vi "IMAQdx_AbsImage_Flea3_v4.4.vi"() -> ()   [LabVIEW 2012]
doc: "Take a single PixelFly exposure and display the result as an intensity graph.This VI illustrates the basics of taking an exposure with the PixelFly camera. Use Ctrl-H to get help on any of the controls\n\nCopyright 2001, The Cooke Corporation."
uses:
  LabVIEW Data V4.10/Shared Libraries/Controls/FileName_Cluster.ctl
  <vilib>/userdefined/High Color/IMAQdx.ctl
  <vilib>/vision/driver/IMAQdx.llb/IMAQdx Acquisition Mode.ctl
  Shared Libraries/Controls/FileInfo_Global.vi
  <vilib>/vision/driver/NI_Vision_Acquisition_Software.lvlib
panel:
  out "DDE Done":bool=TRUE
  out "Waiting for PIXIS file":bool=TRUE
  in  "Flea Acquire":bool=TRUE
  in  "PIXIS Acquire":bool=TRUE
  out "PIXIS Loop":i32
  out "CycleDone":bool
  out "PIXIS Frames":i64
  in  "Interrupt":bool
  out "Status":string="Running..."
  in  "stop":bool
  in  "Tab Control":enum32{"Setup", "Images", "Hardware status"}(tab)=enum."Images"
  in  "PIXIS Data Series Name":string="Sr_PIXIS_Seq"
  in  "Flea File Parameters":T1={"Data Root"=path "C:/Experiment/Data", "Index"=4, "Instrument"="Flea3_20S4M"} {"Index" format="%04d"}
  in  "PIXIS Wave Name":string="Test_Img"
  out "PIXIS Image Note":string="Experiment=Sr\nCamera_ID=PIXIS\nImageType=Raw\nDataType=Absorption\nImageDirection=XY\nMagnification=5.480000E+0\nFileNumber=4\nIndex=0\nIndexedWaves=BlueLaserLockOffset;DipPowX;DipPowX2;DipPowZ;DoppCoolDet;DoppCoolSweep;Nspacers;Pdet;TOF;TOFaux;Xshim;Yshim;ZshimVar;bLoadT;bMapT;combWidthI;dopCoolT;freq;holdT;loadT;rMOTbroadDetuningF;rMOTbroadDetuningI;rMOTpow2;rMOTpow3;rMOTpow4;singleFreqDet;varWaveP1\nIndexedValues=525.000000000000E-3;3.00000000000000E+0;3.00000000000000E+0;250.000000000000E-3;-1.78000000000000E+3;20.0000000000000E+0;4.00000000000000E+0;600.000000000000E-3;25.0000000000000E-3;18.0000000000000E-3;350.000000000000E-3;875.000000000000E-3;1.52200000000000E+0;5.40000000000000E+0;400.000000000000E-6;2.25000000000000E+0;20.0000000000000E-3;3.00000000000000E+3;500.000000000000E-3;35.0000000000000E-3;2.22500000000000E+0;2.45000000000000E+0;1.60000000000000E+0;1.35000000000000E+0;1.30000000000000E+0;-1.57500000000000E+3;3.50000000000000E+0\n# Current Variables\n#\nholdT = 5.000000E-1\nBlueLaserLockOffset = 5.250000E-1\nDipPowX = 3.000000E+0\nDipPowX2 = 3.000000E+0\nDipPowXLat = 1.500000E+0\nDipPowZ = 2.500000E-1\nDipPowZ2 = 2.500000E-2\nDipPowZ3 = 2.500000E-2\nDoppCoolDet = -1.780000E+3\nDoppCoolSweep = 2.000000E+1\nHeatingAmp = 1.000000E-1\nMOTPow = 8.000000E+0\nMOTcurrent = -7.500000E+0\nMOTdetuning = -4.500000E+1\nNspacers = 4.000000E+0\nPdet = 6.000000E-1\nPdet2 = 5.000000E-2\nProbeDet = 0.000000E+0\nProbePow = 2.000000E+0\nTOF = 2.500000E-2\nTOFaux = 1.800000E-2\nXshim = 3.500000E-1\nYshim = 8.750000E-1\nZshim = 1.600000E+0\nZshimVar = 1.522000E+0\nbLoadT = 5.400000E+0\nbMapT = 4.000000E-4\ncombWidthF = 1.500000E-1\ncombWidthI = 2.250000E+0\ncompensation = -3.981000E+0\ndopCoolT = 2.000000E-2\ndopCoolT1 = 1.500000E-2\nfreq = 3.000000E+3\nloadT = 3.500000E-2\nminus_zman = -7.904000E+0\nplus_zman = -9.792000E+0\nrMOTbroadDetuningF = 2.225000E+0\nrMOTbroadDetuningI = 2.450000E+0\nrMOTcurrF = -2.000000E-1\nrMOTcurrI = -2.000000E-1\nrMOTpow1 = 7.000000E+0\nrMOTpow2 = 1.600000E+0\nrMOTpow3 = 1.350000E+0\nrMOTpow4 = 1.300000E+0\nsingleFreqDet = -1.575000E+3\ntEvap0 = 1.000000E-1\ntEvap1 = 2.000000E+0\ntEvap2 = 3.000000E-1\ntau = 6.000000E-1\nvarWaveP1 = 3.500000E+0\nvarWaveP2 = 3.500000E+0\n#\n# Master Staging List\n#Comment\tMarker\tMode\tGroup\tDelay\tX ODT Shuttter\tX ODT AO TTL\tY ODT Shutter\tY ODT AO TTL\tZ ODT Shutter\tZ ODT AO TTL\t707 Shutter\tPB_7\tPB_8\tFreq Switch rMOT\trMOT AO TTL\t\tTrans AO TTL\tProbe AO TTL\tZman AO TTL\tbMOT AO TTL\t60 Hz Trig Gate\tWindow Heater TTL\tPB_18\tPB_19\tPB_20 Trigger Dev3\tPB_21 Trigger Dev2\tPB_22 Trigger Dev1\tPB_23 Trigger Dev0\tStep\t~Atomic Beam Shutter\tGate Valve\tDO0_2\tDO0_3\t~Zman Coils\t~ MOT Coils\t~ Dipole Flea3 Shutter\trMOT Shutter\t+Zeeman Coils\t-Zeeman Coils\tCompensation Coils\tMOT Coils\trMOT AO Power\trMOT Freq Amplitude\trMOT Freq Offset\tAO0_7\tTrans Shutter\tProbe Shutter\tZman Shutter\tbMOT Shutter\tDO1_4\t679 Shutter\t~ Pixis Shutter\t~Abs Flea3 Shutter\tMOT AO Frequency\tMOT AO Power\tProbe AO Power\tProbe AO Frequency\tX Shim Coils\tY Shim Coils\tZ Shim Coils\tZ ODT AO Power\tPIXIS Ext Shutter\tD02_1\tD02_2\tD02_3\tD02_4\tD02_5\tD02_6\tD02_7\tAO2_0\tAO2_1\tD03_0\tD03_1\tD03_2\tD03_3\tD03_4\tD03_5\tD03_6\tD03_7\tAO3_0\tAO3_1\tAO3_2\tVariable Waveplate\t461 Spec Offset\tAO3_5\tAO3_6\tX ODT AO Power\tSRS Freq\tSRS Amp\tSRS Offset\tSRS Func Type\tRedMotDDS\tRedMotDDS_ 0\tRedMotDDS_ 1\tRedMotDDS_ 2\r\n\r\nreset\t\tRamp\t1\t.1\t1\t1\t0\t0\t0\t1\t1\t0\t0\t0\t1\t0\t1\t1\t1\t0\t0\t0\t0\t0\t0\t0\t0\t0\t0\t0\t1\t0\t0\t0\t0\t1\t0\tplus_zman\tminus_zman\tcompensation\tMOTcurrent\trMOTpow1\tcombAmplitude(combWidthI)\trMOTdelta(-(rMOTbroadDetuningI +combWidthI/2))\t0\t1\t0\t1\t1\t0\t1\t1\t1\tbMOTdelta(MOTdetuning)\tbMOTpow(0.5)\tProbePow\tPdet2\tXshim\tYshim\tZshim\tODTpowY(DipPowZ)\t0\t0\t0\t0\t0\t0\t0\t0\t0\t0\t0\t0\t0\t0\t0\t0\t0\t0\t0\t0\t0\tvarWaveP1\tBlueLaserLockOffset\t0\t0\tODTpowX(DipPowX)\tfreq\tHeatingAmp\t0\tSine\tDetuning\tsingleFreqDet\t-20\t8\r\nblue MOT load\t\tRamp\t1\tbLoadT\t1\t1\t0\t0\t0\t1\t0\t0\t0\t0\t1\t0\t1\t1\t1\t1\t0\t0\t0\t0\t0\t0\t0\t0\t0\t0\t1\t0\t0\t0\t0\t1\t0\tplus_zman\tminus_zman\tcompensation\tMOTcurrent\trMOTpow1\tcombAmplitude(combWidthI)\trMOTdelta(-(rMOTbroadDetuningI +combWidthI/2))\t0\t1\t0\t1\t1\t0\t0\t1\t1\tbMOTdelta(MOTdetuning)\tbMOTpow(MOTPow)\tProbePow\tPdet2\tXshim\tYshim\tZshim\tODTpowY(DipPowZ)\t0\t0\t0\t0\t0\t0\t0\t0\t0\t0\t0\t0\t0\t0\t0\t0\t0\t0\t0\t0\t0\tvarWaveP1\tBlueLaserLockOffset\t0\t0\tODTpowX(DipPowX)\tfreq\tHeatingAmp\t0\tSine\tDetuning\tsingleFreqDet\t-20\t8\r\npretrig\t\tRamp\t1\t6.244e-3\t1\t1\t0\t0\t0\t1\t0\t0\t0\t0\t1\t0\t1\t1\t1\t1\t0\t1\t0\t0\t0\t0\t0\t0\t0\t0\t1\t0\t0\t0\t0\t0\t0\tplus_zman\tminus_zman\tcompensation\tMOTcurrent\trMOTpow1\tcombAmplitude(combWidthI)\trMOTdelta(-(rMOTbroadDetuningI +combWidthI/2))\t0\t1\t0\t1\t1\t0\t0\t0\t0\tbMOTdelta(MOTdetuning)\tbMOTpow(MOTPow)\tProbePow\tPdet2\tXshim\tYshim\tZshim\tODTpowY(DipPowZ)\t0\t0\t0\t0\t0\t0\t0\t0\t0\t0\t0\t0\t0\t0\t0\t0\t0\t0\t0\t0\t0\tvarWaveP1\tBlueLaserLockOffset\t0\t0\tODTpowX(DipPowX)\tfreq\tHeatingAmp\t0\tSine\tDetuning\tsingleFreqDet\t-20\t8\r\nCamWaitTime\t\tRamp\t1\t0.275\t1\t1\t0\t0\t0\t1\t0\t0\t0\t0\t1\t0\t1\t1\t1\t1\t0\t1\t0\t0\t0\t0\t0\t0\t0\t0\t1\t0\t0\t0\t0\t1\t0\tplus_zman\tminus_zman\tcompensation\tMOTcurrent\trMOTpow1\tcombAmplitude(combWidthI)\trMOTdelta(-(rMOTbroadDetuningI +combWidthI/2))\t0\t1\t0\t1\t1\t0\t0\t1\t1\tbMOTdelta(MOTdetuning)\tbMOTpow(MOTPow)\tProbePow\tPdet2\tXshim\tYshim\tZshim\tODTpowZ(DipPowZ)\t0\t0\t0\t0\t0\t0\t0\t0\t0\t0\t0\t0\t0\t0\t0\t0\t0\t0\t0\t0\t0\tvarWaveP1\tBlueLaserLockOffset\t0\t0\tODTpowX(DipPowX)\tfreq\tHeatingAmp\t0\tSine\tDetuning\tsingleFreqDet\t-20\t8\r\nProbeShutOn\t\tRamp\t1\t1120e-6\t1\t1\t0\t0\t0\t1\t0\t0\t0\t0\t1\t0\t1\t1\t1\t1\t0\t1\t0\t0\t0\t0\t0\t0\t0\t0\t1\t0\t0\t0\t0\t1\t1\tplus_zman\tminus_zman\tcompensation\tMOTcurrent\trMOTpow1\tcombAmplitude(combWidthI)\trMOTdelta(-(rMOTbroadDetuningI +combWidthI/2))\t0\t1\t0\t1\t1\t0\t0\t1\t1\tbMOTdelta(MOTdetuning)\tbMOTpow(MOTPow)\tProbePow\tPdet2\tXshim\tYshim\tZshim\tODTpowZ(DipPowZ)\t0\t0\t0\t0\t0\t0\t0\t0\t0\t0\t0\t0\t0\t0\t0\t0\t0\t0\t0\t0\t0\tvarWaveP1\tBlueLaserLockOffset\t0\t0\tODTpowX(DipPowX)\tfreq\tHeatingAmp\t0\tSine\tDetuning\tsingleFreqDet\t-20\t8\r\nRepumpShutOff\t\tRamp\t1\t260e-6\t1\t1\t0\t0\t0\t1\t0\t0\t0\t0\t1\t0\t1\t1\t1\t1\t0\t1\t0\t0\t0\t0\t0\t0\t0\t0\t1\t0\t0\t0\t0\t1\t1\tplus_zman\tminus_zman\tcompensation\tMOTcurrent\trMOTpow1\tcombAmplitude(combWidthI)\trMOTdelta(-(rMOTbroadDetuningI +combWidthI/2))\t0\t1\t0\t0\t1\t0\t0\t1\t1\tbMOTdelta(MOTdetuning)\tbMOTpow(MOTPow)\tProbePow\tPdet2\tXshim\tYshim\tZshim\tODTpowZ(DipPowZ)\t0\t0\t0\t0\t0\t0\t0\t0\t0\t0\t0\t0\t0\t0\t0\t0\t0\t0\t0\t0\t0\tvarWaveP1\tBlueLaserLockOffset\t0\t0\tODTpowX(DipPowX)\tfreq\tHeatingAmp\t0\tSine\tDetuning\tsingleFreqDet\t-20\t8\r\nMOTShutOff\t\tRamp\t1\t1370e-6\t1\t1\t0\t0\t0\t1\t1\t0\t0\t0\t1\t0\t1\t1\t1\t1\t0\t1\t0\t0\t0\t0\t0\t0\t0\t0\t1\t0\t0\t0\t0\t1\t1\tplus_zman\tminus_zman\tcompensation\tMOTcurrent\trMOTpow1\tcombAmplitude(combWidthI)\trMOTdelta(-(rMOTbroadDetuningI +combWidthI/2))\t0\t1\t0\t0\t0\t0\t1\t1\t1\tbMOTdelta(MOTdetuning)\tbMOTpow(MOTPow)\tProbePow\tPdet2\tXshim\tYshim\tZshim\t0\t0\t0\t0\t0\t0\t0\t0\t0\t0\t0\t0\t0\t0\t0\t0\t0\t0\t0\t0\t0\t0\tvarWaveP1\tBlueLaserLockOffset\t0\t0\tODTpowX(DipPowX)\tfreq\tHeatingAmp\t0\tSine\tDetuning\tsingleFreqDet\t-20\t8\r\nCoil Switch\t\tRamp\t1\t220e-6\t1\t1\t0\t0\t0\t0\t1\t0\t0\t0\t1\t0\t1\t1\t0\t0\t0\t1\t0\t0\t0\t0\t0\t0\t0\t0\t1\t0\t0\t0\t0\t1\t1\tplus_zman\tminus_zman\tcompensation\trMOTcurrI\trMOTpow1\tcombAmplitude(combWidthI)\trMOTdelta(-(rMOTbroadDetuningI +combWidthI/2))\t0\t1\t0\t0\t0\t0\t1\t1\t1\tbMOTdelta(MOTdetuning)\tbMOTpow(0.5)\tProbePow\tPdet2\tXshim\tYshim\tZshim\t0\t0\t0\t0\t0\t0\t0\t0\t0\t0\t0\t0\t0\t0\t0\t0\t0\t0\t0\t0\t0\t0\tvarWaveP1\tBlueLaserLockOffset\t0\t0\tODTpowX(DipPowX)\tfreq\tHeatingAmp\t0\tSine\tDetuning\tsingleFreqDet\t-20\t8\r\n60HzTrigger\t\tHalt\t1\t10u\t1\t1\t0\t0\t0\t0\t1\t0\t0\t0\t1\t0\t1\t1\t0\t0\t1\t1\t0\t0\t0\t0\t0\t0\t0\t0\t1\t0\t0\t0\t0\t1\t1\tplus_zman\tminus_zman\tcompensation\trMOTcurrI\trMOTpow1\tcombAmplitude(combWidthI)\trMOTdelta(-(rMOTbroadDetuningI +combWidthI/2))\t0\t1\t0\t0\t0\t0\t1\t1\t1\tbMOTdelta(MOTdetuning)\tbMOTpow(0.5)\tProbePow\tPdet2\tXshim\tYshim\tZshim\t0\t0\t0\t0\t0\t0\t0\t0\t0\t0\t0\t0\t0\t0\t0\t0\t0\t0\t0\t0\t0\t0\tvarWaveP1\tBlueLaserLockOffset\t0\t0\tODTpowX(DipPowX)\tfreq\tHeatingAmp\t0\tSine\tDetuning\tsingleFreqDet\t-20\t8\r\nCapture Red MOT\t\tRamp\t1\t.1\t1\t1\t0\t0\t0\t0\t1\t0\t0\t0\t1\t0\t0\t1\t0\t0\t0\t1\t0\t0\t0\t0\t0\t0\t0\t0\t1\t0\t0\t0\t0\t1\t1\tplus_zman\tminus_zman\tcompensation\trMOTcurrI\trMOTpow1\tcombAmplitude(combWidthI)\trMOTdelta(-(rMOTbroadDetuningI +combWidthI/2))\t0\t1\t0\t0\t0\t0\t1\t1\t1\tbMOTdelta(MOTdetuning)\tbMOTpow(0.5)\tProbePow\tPdet2\tXshim\tYshim\tZshim\tODTpowZ(DipPowZ)\t0\t0\t0\t0\t0\t0\t0\t0\t0\t0\t0\t0\t0\t0\t0\t0\t0\t0\t0\t0\t0\tvarWaveP1\tBlueLaserLockOffset\t0\t0\tODTpowX(DipPowX)\tfreq\tHeatingAmp\t0\tSine\tDetuning\tsingleFreqDet\t-20\t8\r\nRamp Red MOT\t\tRamp\t1\t.4\t1\t1\t0\t0\t0\t0\t1\t0\t0\t0\t1\t0\t0\t1\t0\t0\t0\t1\t0\t0\t0\t0\t0\t0\t10u\t0\t1\t0\t0\t0\t0\t1\t1\tplus_zman\tminus_zman\tcompensation\trMOTcurrI\tHalfGaussRamp(t,rMOTpow1,rMOTpow2, .4)\tLineRamp(f,combAmplitude(combWidthI),combAmplitude(combWidthF))\tLineRamp(f,rMOTdelta(-(rMOTbroadDetuningI +combWidthI/2)),rMOTdelta(-(rMOTbroadDetuningF +combWidthF/2)))\t0\t1\t0\t0\t0\t0\t1\t1\t1\tbMOTdelta(MOTdetuning)\tbMOTpow(0.5)\tProbePow\tPdet2\tXshim\tYshim\tLineRamp(f,Zshim,ZshimVar)\tODTpowZ(DipPowZ)\t0\t0\t0\t0\t0\t0\t0\t0\t0\t0\t0\t0\t0\t0\t0\t0\t0\t0\t0\t0\t0\tvarWaveP1\tLineRamp(f,BlueLaserLockOffset,Pdet)\t0\t0\tODTpowX(DipPowX)\tfreq\tHeatingAmp\t0\tSine\tDetuning\tsingleFreqDet\t-20\t8\r\nSF\t\tRamp\t1\t.07\t1\t1\t0\t0\t0\t0\t0\t0\t0\t1\t1\t0\t0\t1\t0\t0\t0\t1\t0\t0\t0\t0\t0\t0\t10u\t0\t1\t0\t0\t0\t0\t1\t1\tplus_zman\tminus_zman\tcompensation\trMOTcurrI\tLineRamp(f,rMOTpow2,rMOTpow3)\tcombAmplitude(combWidthF)\trMOTdelta(-(rMOTbroadDetuningF +combWidthF/2))\t0\t1\t0\t0\t0\t0\t0\t1\t1\tbMOTdelta(MOTdetuning)\tbMOTpow(0.5)\tProbePow\tPdet2\tXshim\tYshim\tZshimVar\tODTpowZ(DipPowZ)\t0\t0\t0\t0\t0\t0\t0\t0\t0\t0\t0\t0\t0\t0\t0\t0\t0\t0\t0\t0\t0\tvarWaveP1\tPdet\t0\t0\tODTpowX(DipPowX)\tfreq\tHeatingAmp\t0\tSine\tDetuning\tsingleFreqDet\t-20\t8\r\nload1\t\tRamp\t1\tloadT\t1\t1\t0\t0\t0\t0\t0\t0\t0\t1\t1\t0\t0\t1\t0\t0\t0\t1\t0\t0\t0\t0\t0\t0\t0\t0\t1\t0\t0\t0\t0\t1\t1\tplus_zman\tminus_zman\tcompensation\trMOTcurrI\trMOTpow3\tcombAmplitude(combWidthF)\trMOTdelta(-(rMOTbroadDetuningF +combWidthF/2))\t0\t1\t0\t0\t0\t0\t0\t1\t1\tbMOTdelta(MOTdetuning)\tbMOTpow(0.5)\tProbePow\tPdet2\tXshim\tYshim\tZshimVar\tODTpowZ(DipPowZ)\t0\t0\t0\t0\t0\t0\t0\t0\t0\t0\t0\t0\t0\t0\t0\t0\t0\t0\t0\t0\t0\tvarWaveP1\tPdet\t0\t0\tODTpowX(DipPowX)\tfreq\tHeatingAmp\t0\tSine\tDetuning\tsingleFreqDet\t-20\t8\r\nload2\t\tRamp\t0\t.05\t1\t1\t0\t0\t0\t0\t0\t0\t0\t1\t1\t0\t0\t1\t0\t0\t0\t1\t0\t0\t0\t0\t0\t0\t0\t0\t1\t0\t0\t0\t0\t1\t1\tplus_zman\tminus_zman\tcompensation\trMOTcurrI\trMOTpow3\tcombAmplitude(combWidthF)\trMOTdelta(-(rMOTbroadDetuningF +combWidthF/2))\t0\t1\t0\t0\t0\t0\t0\t1\t1\tbMOTdelta(MOTdetuning)\tbMOTpow(0.5)\tProbePow\tPdet2\tXshim\tYshim\tZshimVar\tODTpowZ(DipPowZ)\t0\t0\t0\t0\t0\t0\t0\t0\t0\t0\t0\t0\t0\t0\t0\t0\t0\t0\t0\t0\t0\tvarWaveP1\tPdet\t0\t0\tODTpowX(DipPowX)\tfreq\tHeatingAmp\t0\tSine\tDetuning\tsingleFreqDet\t-20\t8\r\ndrop Red MOT\t\tRamp\t1\t.05\t1\t1\t0\t0\t0\t0\t0\t0\t0\t1\t0\t0\t0\t1\t0\t0\t0\t1\t0\t0\t0\t0\t0\t0\t0\t0\t1\t0\t0\t0\t1\t1\t0\tplus_zman\tminus_zman\tcompensation\trMOTcurrF\trMOTpow3\tcombAmplitude(combWidthF)\trMOTdelta(-(rMOTbroadDetuningF +combWidthF/2))\t0\t1\t0\t0\t0\t0\t0\t1\t1\tbMOTdelta(MOTdetuning)\tbMOTpow(0.5)\tProbePow\tPdet2\tXshim\tYshim\tZshimVar\tODTpowZ(DipPowZ)\t0\t0\t0\t0\t0\t0\t0\t0\t0\t0\t0\t0\t0\t0\t0\t0\t0\t0\t0\t0\t0\tvarWaveP1\tPdet\t0\t0\tODTpowX(DipPowX)\tfreq\tHeatingAmp\t0\tSine\tDetuning\tsingleFreqDet\t-20\t8\r\nramp Trap\t\tRamp\t0\t.05\t1\t1\t0\t0\t0\t0\t0\t0\t0\t1\t0\t0\t0\t1\t0\t0\t0\t1\t0\t0\t0\t0\t0\t0\t10u\t0\t1\t0\t0\t0\t1\t1\t0\tplus_zman\tminus_zman\tcompensation\trMOTcurrF\trMOTpow3\tcombAmplitude(combWidthF)\trMOTdelta(-(rMOTbroadDetuningF +combWidthF/2))\t0\t1\t0\t0\t0\t0\t0\t1\t1\tbMOTdelta(MOTdetuning)\tbMOTpow(0.5)\tProbePow\tPdet2\tXshim\tYshim\tZshimVar\tODTpowZ(DipPowZ)\t0\t0\t0\t0\t0\t0\t0\t0\t0\t0\t0\t0\t0\t0\t0\t0\t0\t0\t0\t0\t0\tvarWaveP1\tPdet\t0\t0\tSinRamp(t,(ODTpowX(DipPowX)+ODTpowX(DipPowX2))/2,(ODTpowX(DipPowX2)-ODTpowX(DipPowX))/2,10,3*pi/2)\tfreq\tHeatingAmp\t0\tSine\tDetuning\tsingleFreqDet\t-20\t8\r\nhold\t\tRamp\t0\t.01\t1\t1\t0\t0\t0\t0\t0\t0\t0\t1\t0\t0\t0\t1\t0\t0\t0\t1\t0\t0\t0\t0\t0\t0\t0\t0\t1\t0\t0\t0\t1\t1\t1\tplus_zman\tminus_zman\tcompensation\trMOTcurrF\trMOTpow4\tcombAmplitude(combWidthF)\trMOTdelta(-(rMOTbroadDetuningF +combWidthF/2))\t0\t1\t0\t0\t0\t0\t0\t1\t1\tbMOTdelta(MOTdetuning)\tbMOTpow(0.5)\tProbePow\tPdet2\tXshim\tYshim\tZshimVar\tODTpowZ(DipPowZ)\t0\t0\t0\t0\t0\t0\t0\t0\t0\t0\t0\t0\t0\t0\t0\t0\t0\t0\t0\t0\t0\tvarWaveP1\tPdet\t0\t0\tODTpowX(DipPowX2)\tfreq\tHeatingAmp\t0\tSine\tDetuning\tDoppCoolDet\t-20\t8\r\nDoppler Cool1\t\tRamp\t0\tdopCoolT\t1\t1\t0\t0\t0\t0\t0\t0\t0\t1\t1\t0\t0\t1\t0\t0\t0\t1\t0\t0\t0\t0\t0\t0\t10u\t0\t1\t0\t0\t0\t1\t1\t1\tplus_zman\tminus_zman\tcompensation\trMOTcurrF\trMOTpow4\tcombAmplitude(combWidthF)\trMOTdelta(-(rMOTbroadDetuningF +combWidthF/2))\t0\t0\t0\t0\t0\t0\t0\t1\t1\tbMOTdelta(MOTdetuning)\tbMOTpow(0.5)\tProbePow\tPdet2\tXshim\tYshim\tZshimVar\tODTpowZ(DipPowZ)\t0\t0\t0\t0\t0\t0\t0\t0\t0\t0\t0\t0\t0\t0\t0\t0\t0\t0\t0\t0\t0\tvarWaveP1\tPdet\t0\t0\tODTpowX(DipPowX2)\tfreq\tHeatingAmp\t0\tSine\tDetuning\tDoppCoolDet\t-20\t8\r\nDoppler Cool2\t\tRamp\t0\tdopCoolT\t1\t1\t0\t0\t0\t0\t0\t0\t0\t1\t1\t0\t0\t1\t0\t0\t0\t1\t0\t0\t0\t0\t0\t0\t10u\t0\t1\t0\t0\t0\t1\t1\t1\tplus_zman\tminus_zman\tcompensation\trMOTcurrF\trMOTpow4\tcombAmplitude(combWidthF)\trMOTdelta(-(rMOTbroadDetuningF +combWidthF/2))\t0\t0\t0\t0\t0\t0\t0\t1\t1\tbMOTdelta(MOTdetuning)\tbMOTpow(0.5)\tProbePow\tPdet2\tXshim\tYshim\tZshimVar\tODTpowZ(DipPowZ)\t0\t0\t0\t0\t0\t0\t0\t0\t0\t0\t0\t0\t0\t0\t0\t0\t0\t0\t0\t0\t0\tvarWaveP1\tPdet\t0\t0\tODTpowX(DipPowX2)\tfreq\tHeatingAmp\t0\tSine\tRamp\tDoppCoolDet\tDoppCoolDet-DoppCoolSweep\tdopCoolT*1000\r\nDoppler Cool3\t\tRamp\t0\tdopCoolT\t1\t1\t0\t0\t0\t0\t0\t0\t0\t1\t1\t0\t0\t1\t0\t0\t0\t1\t0\t0\t0\t0\t0\t0\t10u\t0\t1\t0\t0\t0\t1\t1\t1\tplus_zman\tminus_zman\tcompensation\trMOTcurrF\trMOTpow4\tcombAmplitude(combWidthF)\trMOTdelta(-(rMOTbroadDetuningF +combWidthF/2))\t0\t0\t0\t0\t0\t0\t0\t1\t1\tbMOTdelta(MOTdetuning)\tbMOTpow(0.5)\tProbePow\tPdet2\tXshim\tYshim\tZshimVar\tODTpowZ(DipPowZ)\t0\t0\t0\t0\t0\t0\t0\t0\t0\t0\t0\t0\t0\t0\t0\t0\t0\t0\t0\t0\t0\tvarWaveP1\tPdet\t0\t0\tODTpowX(DipPowX2)\tfreq\tHeatingAmp\t0\tSine\tDetuning\tDoppCoolDet-DoppCoolSweep\tDoppCoolDet-DoppCoolSweep\tdopCoolT*1000\r\nhold\t\tRamp\t0\tholdT\t1\t1\t0\t0\t0\t0\t0\t0\t0\t1\t0\t0\t0\t1\t0\t0\t0\t1\t0\t0\t0\t0\t0\t0\t0\t0\t1\t0\t0\t0\t1\t1\t0\tplus_zman\tminus_zman\tcompensation\trMOTcurrF\trMOTpow4\tcombAmplitude(combWidthF)\trMOTdelta(-(rMOTbroadDetuningF +combWidthF/2))\t0\t1\t0\t0\t0\t0\t0\t1\t1\tbMOTdelta(MOTdetuning)\tbMOTpow(0.5)\tProbePow\tPdet2\tXshim\tYshim\tZshimVar\tODTpowZ(DipPowZ)\t0\t0\t0\t0\t0\t0\t0\t0\t0\t0\t0\t0\t0\t0\t0\t0\t0\t0\t0\t0\t0\tvarWaveP1\tPdet\t0\t0\tODTpowX(DipPowX2)\tfreq\tHeatingAmp\t0\tSine\tDetuning\tDoppCoolDet-DoppCoolSweep\tDoppCoolDet-DoppCoolSweep\tdopCoolT*1000\r\ndrop HTrap\t\tRamp\t0\t.03\t1\t1\t0\t0\t1\t1\t1\t0\t0\t1\t0\t0\t0\t1\t0\t0\t0\t1\t0\t0\t0\t0\t0\t0\t0\t0\t1\t0\t0\t0\t0\t1\t0\tplus_zman\tminus_zman\tcompensation\trMOTcurrF\trMOTpow3\tcombAmplitude(combWidthF)\trMOTdelta(-(rMOTbroadDetuningF +combWidthF/2))\t0\t1\t0\t0\t0\t0\t1\t1\t1\tbMOTdelta(MOTdetuning)\tbMOTpow(0.5)\tProbePow\tPdet2\tXshim\tYshim\tZshimVar\tODTpowZ(DipPowZ)\t0\t0\t0\t0\t0\t0\t0\t0\t0\t0\t0\t0\t0\t0\t0\t0\t0\t0\t0\t0\t0\tvarWaveP1\tPdet\t0\t0\tODTpowX(DipPowX)\tfreq\tHeatingAmp\t0\tSine\tDetuning\tsingleFreqDet\tDoppCoolDet-DoppCoolSweep\tdopCoolT*1000\r\nmodulate\t\tRamp\t0\t3m\t1\t1\t0\t0\t1\t1\t1\t0\t0\t1\t0\t0\t0\t1\t0\t0\t0\t1\t0\t0\t0\t0\t0\t0\t0\t0\t1\t0\t0\t0\t0\t1\t0\tplus_zman\tminus_zman\tcompensation\trMOTcurrF\trMOTpow3\tcombAmplitude(combWidthF)\trMOTdelta(-(rMOTbroadDetuningF +combWidthF/2))\t0\t1\t0\t0\t0\t0\t1\t1\t1\tbMOTdelta(MOTdetuning)\tbMOTpow(0.5)\tProbePow\tPdet2\tXshim\tYshim\tZshimVar\tODTpowZ(DipPowZ)\t0\t0\t0\t0\t0\t0\t0\t0\t0\t0\t0\t0\t0\t0\t0\t0\t0\t0\t0\t0\t0\tvarWaveP1\tPdet\t0\t0\tODTpowX(DipPowX)\tfreq\tHeatingAmp\t0\tSine\tDetuning\tsingleFreqDet\tDoppCoolDet-DoppCoolSweep\tdopCoolT*1000\r\nEvaporation\t\tRamp\t0\ttEvap1\t1\t1\t0\t0\t1\t1\t1\t0\t0\t1\t0\t0\t0\t1\t0\t0\t0\t1\t0\t0\t0\t0\t0\t0\t1m\t0\t1\t0\t0\t0\t0\t1\t0\tplus_zman\tminus_zman\tcompensation\trMOTcurrF\trMOTpow3\tcombAmplitude(combWidthF)\trMOTdelta(-(rMOTbroadDetuningF +combWidthF/2))\t0\t1\t0\t0\t0\t0\t1\t1\t1\tbMOTdelta(MOTdetuning)\tbMOTpow(0.5)\tProbePow\tPdet2\tXshim\tYshim\tZshimVar\tODTpowZ(DipPowZ)\t0\t0\t0\t0\t0\t0\t0\t0\t0\t0\t0\t0\t0\t0\t0\t0\t0\t0\t0\t0\t0\tvarWaveP1\tPdet\t0\t0\tExpRamp2(t,0,ODTpowX(DipPowX),ODTpowX(DipPowX2),tau)\tfreq\tHeatingAmp\t0\tSine\tDetuning\tsingleFreqDet\tDoppCoolDet-DoppCoolSweep\tdopCoolT*1000\r\ndrop\t\tRamp\t0\t.01\t1\t1\t0\t0\t1\t1\t1\t0\t0\t1\t0\t0\t0\t1\t0\t0\t0\t1\t0\t0\t0\t0\t0\t0\t0\t0\t1\t0\t0\t0\t0\t1\t0\tplus_zman\tminus_zman\tcompensation\trMOTcurrF\trMOTpow3\tcombAmplitude(combWidthF)\trMOTdelta(-(rMOTbroadDetuningF +combWidthF/2))\t0\t1\t0\t0\t0\t0\t1\t1\t1\tbMOTdelta(MOTdetuning)\tbMOTpow(0.5)\tProbePow\tPdet2\tXshim\tYshim\tZshimVar\tODTpowZ(DipPowZ)\t0\t0\t0\t0\t0\t0\t0\t0\t0\t0\t0\t0\t0\t0\t0\t0\t0\t0\t0\t0\t0\tvarWaveP2\tPdet\t0\t0\tODTpowX(DipPowXLat)\tfreq\tHeatingAmp\t0\tSine\tDetuning\tsingleFreqDet\tDoppCoolDet-DoppCoolSweep\tdopCoolT*1000\r\nband map\t\tRamp\t0\tbMapT\t1\t1\t0\t0\t1\t1\t1\t0\t0\t1\t0\t0\t0\t1\t0\t0\t0\t1\t0\t0\t0\t0\t0\t0\t2u\t0\t1\t0\t0\t0\t0\t1\t0\tplus_zman\tminus_zman\tcompensation\trMOTcurrF\trMOTpow3\tcombAmplitude(combWidthF)\trMOTdelta(-(rMOTbroadDetuningF +combWidthF/2))\t0\t1\t0\t0\t0\t0\t1\t1\t1\tbMOTdelta(MOTdetuning)\tbMOTpow(0.5)\tProbePow\tPdet2\tXshim\tYshim\tZshimVar\tLineRamp(f,ODTpowZ(DipPowZ),ODTpowZ(-0.2))\t0\t0\t0\t0\t0\t0\t0\t0\t0\t0\t0\t0\t0\t0\t0\t0\t0\t0\t0\t0\t0\tvarWaveP2\tPdet\t0\t0\tLineRamp(f,ODTpowX(DipPowX),0)\tfreq\tHeatingAmp\t0\tSine\tDetuning\tsingleFreqDet\tDoppCoolDet-DoppCoolSweep\tdopCoolT*1000\r\nband map delay\t\tRamp\t0\t10u\t1\t1\t0\t0\t1\t1\t1\t0\t0\t1\t0\t0\t0\t1\t0\t0\t0\t1\t0\t0\t0\t0\t0\t0\t0\t0\t1\t0\t0\t0\t0\t1\t0\tplus_zman\tminus_zman\tcompensation\trMOTcurrF\trMOTpow3\tcombAmplitude(combWidthF)\trMOTdelta(-(rMOTbroadDetuningF +combWidthF/2))\t0\t1\t0\t0\t0\t0\t1\t1\t1\tbMOTdelta(MOTdetuning)\tbMOTpow(0.5)\tProbePow\tPdet2\tXshim\tYshim\tZshimVar\tODTpowZ(DipPowZ)\t0\t0\t0\t0\t0\t0\t0\t0\t0\t0\t0\t0\t0\t0\t0\t0\t0\t0\t0\t0\t0\tvarWaveP2\tPdet\t0\t0\tODTpowX(DipPowXLat)\tfreq\tHeatingAmp\t0\tSine\tDetuning\tsingleFreqDet\tDoppCoolDet-DoppCoolSweep\tdopCoolT*1000\r\nTOF\t\tRamp\t1\tTOFaux\t0\t0\t0\t0\t0\t0\t1\t0\t0\t1\t0\t0\t0\t0\t0\t0\t0\t1\t0\t0\t0\t0\t0\t0\t0\t0\t1\t0\t0\t0\t1\t1\t0\tplus_zman\tminus_zman\tcompensation\trMOTcurrF\trMOTpow4\tcombAmplitude(combWidthF)\trMOTdelta(-(rMOTbroadDetuningF +combWidthF/2))\t0\t1\t1\t0\t0\t0\t1\t1\t1\tbMOTdelta(MOTdetuning)\tbMOTpow(0.5)\tProbePow\tPdet\tXshim\tYshim\tZshimVar\tODTpowZ(DipPowZ)\t1\t0\t0\t0\t0\t0\t0\t0\t0\t0\t0\t0\t0\t0\t0\t0\t0\t0\t0\t0\t0\tvarWaveP2\tPdet\t0\t0\tODTpowX(DipPowX2)\tfreq\tHeatingAmp\t0\tSine\tDetuning\tsingleFreqDet\tDoppCoolDet-DoppCoolSweep\tdopCoolT*1000\r\nTOF\t\tRamp\t1\t.007\t0\t0\t0\t0\t0\t0\t1\t0\t0\t1\t0\t0\t0\t0\t0\t0\t0\t1\t0\t0\t0\t0\t0\t0\t0\t0\t1\t0\t0\t0\t1\t1\t0\tplus_zman\tminus_zman\tcompensation\trMOTcurrF\trMOTpow4\tcombAmplitude(combWidthF)\trMOTdelta(-(rMOTbroadDetuningF +combWidthF/2))\t0\t1\t1\t0\t0\t0\t1\t1\t1\tbMOTdelta(MOTdetuning)\tbMOTpow(0.5)\tProbePow\tPdet\tXshim\tYshim\tZshimVar\tODTpowZ(DipPowZ)\t1\t0\t0\t0\t0\t0\t0\t0\t0\t0\t0\t0\t0\t0\t0\t0\t0\t0\t0\t0\t0\tvarWaveP2\tPdet\t0\t0\tODTpowX(DipPowX2)\tfreq\tHeatingAmp\t0\tSine\tDetuning\tsingleFreqDet\tDoppCoolDet-DoppCoolSweep\tdopCoolT*1000\r\narm FLEA\t\tRamp\t1\t.000044\t0\t0\t0\t0\t0\t0\t1\t0\t0\t1\t0\t0\t0\t0\t0\t0\t0\t0\t0\t0\t0\t0\t0\t0\t0\t0\t1\t0\t0\t0\t1\t0\t0\tplus_zman\tminus_zman\tcompensation\trMOTcurrF\trMOTpow3\tcombAmplitude(combWidthF)\trMOTdelta(-(rMOTbroadDetuningF +combWidthF/2))\t0\t1\t1\t0\t0\t0\t1\t1\t0\tbMOTdelta(MOTdetuning)\tbMOTpow(0.5)\tProbePow\tPdet\tXshim\tYshim\tZshimVar\tODTpowZ(0)\t1\t0\t0\t0\t0\t0\t0\t0\t0\t0\t0\t0\t0\t0\t0\t0\t0\t0\t0\t0\t0\tvarWaveP2\tPdet\t0\t0\tODTpowX(DipPowX)\tfreq\tHeatingAmp\t0\tSine\tDetuning\tsingleFreqDet\tDoppCoolDet-DoppCoolSweep\tdopCoolT*1000\r\natom img\t\tRamp\t1\t10e-6\t0\t0\t0\t0\t0\t0\t1\t0\t0\t1\t0\t0\t0\t1\t0\t0\t0\t0\t0\t0\t0\t0\t0\t0\t0\t0\t1\t0\t0\t0\t1\t0\t0\tplus_zman\tminus_zman\tcompensation\trMOTcurrF\trMOTpow3\tcombAmplitude(combWidthF)\trMOTdelta(-(rMOTbroadDetuningF +combWidthF/2))\t0\t1\t1\t0\t0\t0\t1\t0\t0\tbMOTdelta(MOTdetuning)\tbMOTpow(0.5)\tProbePow\tPdet\tXshim\tYshim\tZshimVar\tODTpowZ(0)\t1\t0\t0\t0\t0\t0\t0\t0\t0\t0\t0\t0\t0\t0\t0\t0\t0\t0\t0\t0\t0\tvarWaveP2\tPdet\t0\t0\tODTpowX(DipPowX)\tfreq\tHeatingAmp\t0\tSine\tDetuning\tsingleFreqDet\tDoppCoolDet-DoppCoolSweep\tdopCoolT*1000\r\natom img\t\tRamp\t0\t2.8e-3\t0\t0\t0\t0\t0\t0\t1\t0\t0\t1\t0\t0\t0\t0\t0\t0\t0\t0\t0\t0\t0\t0\t0\t0\t0\t0\t1\t0\t0\t0\t1\t1\t0\tplus_zman\tminus_zman\tcompensation\trMOTcurrF\trMOTpow3\tcombAmplitude(combWidthF)\trMOTdelta(-(rMOTbroadDetuningF +combWidthF/2))\t0\t1\t1\t0\t0\t0\t1\t1\t1\tbMOTdelta(MOTdetuning)\tbMOTpow(0.5)\tProbePow\tPdet\tXshim\tYshim\tZshimVar\tODTpowZ(DipPowZ)\t1\t0\t0\t0\t0\t0\t0\t0\t0\t0\t0\t0\t0\t0\t0\t0\t0\t0\t0\t0\t0\tvarWaveP2\tPdet\t0\t0\tODTpowX(DipPowX)\tfreq\tHeatingAmp\t0\tSine\tDetuning\tsingleFreqDet\tDoppCoolDet-DoppCoolSweep\tdopCoolT*1000\r\ntransmit img\t\tRamp\t1\t.28\t0\t0\t0\t0\t0\t0\t1\t0\t0\t1\t0\t0\t0\t0\t0\t0\t0\t0\t0\t0\t0\t0\t0\t0\t0\t0\t1\t0\t0\t0\t1\t1\t0\tplus_zman\tminus_zman\tcompensation\trMOTcurrF\trMOTpow3\tcombAmplitude(combWidthF)\trMOTdelta(-(rMOTbroadDetuningF +combWidthF/2))\t0\t1\t1\t0\t0\t0\t1\t1\t1\tbMOTdelta(MOTdetuning)\tbMOTpow(0.5)\tProbePow\tPdet\tXshim\tYshim\tZshimVar\tODTpowZ(DipPowZ)\t1\t0\t0\t0\t0\t0\t0\t0\t0\t0\t0\t0\t0\t0\t0\t0\t0\t0\t0\t0\t0\tvarWaveP2\tPdet\t0\t0\tODTpowX(DipPowX)\tfreq\tHeatingAmp\t0\tSine\tDetuning\tsingleFreqDet\tDoppCoolDet-DoppCoolSweep\tdopCoolT*1000\r\narm PIXIS\t\tRamp\t1\t.007\t1\t1\t0\t0\t0\t1\t1\t0\t0\t1\t1\t0\t0\t0\t1\t1\t0\t0\t0\t0\t0\t0\t0\t0\t0\t0\t1\t0\t0\t0\t1\t1\t0\tplus_zman\tminus_zman\tcompensation\trMOTcurrF\trMOTpow1\tcombAmplitude(combWidthF)\trMOTdelta(-(rMOTbroadDetuningF +combWidthF/2))\t0\t1\t1\t0\t0\t0\t1\t1\t1\tbMOTdelta(MOTdetuning)\tbMOTpow(0.5)\tProbePow\tPdet\tXshim\tYshim\tZshimVar\tODTpowZ(DipPowZ)\t1\t0\t0\t0\t0\t0\t0\t0\t0\t0\t0\t0\t0\t0\t0\t0\t0\t0\t0\t0\t0\tvarWaveP2\tPdet\t0\t0\tODTpowX(DipPowX)\tfreq\tHeatingAmp\t0\tSine\tDetuning\tsingleFreqDet\tDoppCoolDet-DoppCoolSweep\tdopCoolT*1000\r\narm FLEA\t\tRamp\t1\t44e-6\t1\t1\t0\t0\t0\t1\t1\t0\t0\t1\t1\t0\t0\t0\t1\t1\t0\t0\t0\t0\t0\t0\t0\t0\t0\t0\t1\t0\t0\t0\t1\t0\t0\tplus_zman\tminus_zman\tcompensation\trMOTcurrF\trMOTpow1\tcombAmplitude(combWidthF)\trMOTdelta(-(rMOTbroadDetuningF +combWidthF/2))\t0\t1\t1\t0\t0\t0\t1\t1\t0\tbMOTdelta(MOTdetuning)\tbMOTpow(0.5)\tProbePow\tPdet\tXshim\tYshim\tZshimVar\tODTpowZ(DipPowZ)\t1\t0\t0\t0\t0\t0\t0\t0\t0\t0\t0\t0\t0\t0\t0\t0\t0\t0\t0\t0\t0\tvarWaveP2\tPdet\t0\t0\tODTpowX(DipPowX)\tfreq\tHeatingAmp\t0\tSine\tDetuning\tsingleFreqDet\tDoppCoolDet-DoppCoolSweep\tdopCoolT*1000\r\nprobe img\t\tRamp\t1\t10e-6\t1\t1\t0\t0\t0\t1\t1\t0\t0\t1\t1\t0\t0\t1\t1\t1\t0\t0\t0\t0\t0\t0\t0\t0\t0\t0\t1\t0\t0\t0\t1\t0\t0\tplus_zman\tminus_zman\tcompensation\trMOTcurrF\trMOTpow1\tcombAmplitude(combWidthF)\trMOTdelta(-(rMOTbroadDetuningF +combWidthF/2))\t0\t1\t1\t0\t0\t0\t1\t0\t0\tbMOTdelta(MOTdetuning)\tbMOTpow(0.5)\tProbePow\tPdet\tXshim\tYshim\tZshimVar\tODTpowZ(DipPowZ)\t1\t0\t0\t0\t0\t0\t0\t0\t0\t0\t0\t0\t0\t0\t0\t0\t0\t0\t0\t0\t0\tvarWaveP2\tPdet\t0\t0\tODTpowX(DipPowX)\tfreq\tHeatingAmp\t0\tSine\tDetuning\tsingleFreqDet\tDoppCoolDet-DoppCoolSweep\tdopCoolT*1000\r\nprobe img\t\tRamp\t0\t2.8e-3\t1\t1\t0\t0\t0\t1\t1\t0\t0\t1\t1\t0\t0\t0\t1\t1\t0\t0\t0\t0\t0\t0\t0\t0\t0\t0\t1\t0\t0\t0\t1\t1\t0\tplus_zman\tminus_zman\tcompensation\trMOTcurrF\trMOTpow1\tcombAmplitude(combWidthF)\trMOTdelta(-(rMOTbroadDetuningF +combWidthF/2))\t0\t1\t1\t0\t0\t0\t1\t1\t1\tbMOTdelta(MOTdetuning)\tbMOTpow(0.5)\tProbePow\tPdet\tXshim\tYshim\tZshimVar\tODTpowZ(DipPowZ)\t1\t0\t0\t0\t0\t0\t0\t0\t0\t0\t0\t0\t0\t0\t0\t0\t0\t0\t0\t0\t0\tvarWaveP2\tPdet\t0\t0\tODTpowX(DipPowX)\tfreq\tHeatingAmp\t0\tSine\tDetuning\tsingleFreqDet\tDoppCoolDet-DoppCoolSweep\tdopCoolT*1000\r\ntransmit img\t\tRamp\t1\t.28\t1\t1\t0\t0\t0\t1\t1\t0\t0\t1\t1\t0\t0\t0\t1\t1\t0\t0\t0\t0\t0\t0\t0\t0\t0\t0\t1\t0\t0\t0\t1\t1\t0\tplus_zman\tminus_zman\tcompensation\trMOTcurrF\trMOTpow1\tcombAmplitude(combWidthF)\trMOTdelta(-(rMOTbroadDetuningF +combWidthF/2))\t0\t1\t1\t0\t0\t0\t1\t1\t1\tbMOTdelta(MOTdetuning)\tbMOTpow(0.5)\tProbePow\tPdet\tXshim\tYshim\tZshimVar\tODTpowZ(DipPowZ)\t1\t0\t0\t0\t0\t0\t0\t0\t0\t0\t0\t0\t0\t0\t0\t0\t0\t0\t0\t0\t0\tvarWaveP2\tPdet\t0\t0\tODTpowX(DipPowX)\tfreq\tHeatingAmp\t0\tSine\tDetuning\tsingleFreqDet\tDoppCoolDet-DoppCoolSweep\tdopCoolT*1000\r\narm PIXIS\t\tRamp\t1\t.007\t1\t1\t0\t0\t0\t1\t1\t0\t0\t1\t1\t0\t0\t0\t1\t1\t0\t0\t0\t0\t0\t0\t0\t0\t0\t0\t1\t0\t0\t0\t1\t1\t0\tplus_zman\tminus_zman\tcompensation\trMOTcurrF\trMOTpow1\tcombAmplitude(combWidthF)\trMOTdelta(-(rMOTbroadDetuningF +combWidthF/2))\t0\t1\t1\t0\t0\t0\t1\t1\t1\tbMOTdelta(MOTdetuning)\tbMOTpow(0.5)\tProbePow\tPdet\tXshim\tYshim\tZshimVar\tODTpowZ(DipPowZ)\t1\t0\t0\t0\t0\t0\t0\t0\t0\t0\t0\t0\t0\t0\t0\t0\t0\t0\t0\t0\t0\tvarWaveP2\tPdet\t0\t0\tODTpowX(DipPowX)\tfreq\tHeatingAmp\t0\tSine\tDetuning\tsingleFreqDet\tDoppCoolDet-DoppCoolSweep\tdopCoolT*1000\r\narm FLEA\t\tRamp\t1\t44e-6\t1\t1\t0\t0\t0\t1\t1\t0\t0\t1\t1\t0\t0\t0\t1\t1\t0\t0\t0\t0\t0\t0\t0\t0\t0\t0\t1\t0\t0\t0\t1\t0\t0\tplus_zman\tminus_zman\tcompensation\trMOTcurrF\trMOTpow1\tcombAmplitude(combWidthF)\trMOTdelta(-(rMOTbroadDetuningF +combWidthF/2))\t0\t1\t1\t0\t0\t0\t1\t1\t0\tbMOTdelta(MOTdetuning)\tbMOTpow(0.5)\tProbePow\tPdet\tXshim\tYshim\tZshimVar\tODTpowZ(DipPowZ)\t1\t0\t0\t0\t0\t0\t0\t0\t0\t0\t0\t0\t0\t0\t0\t0\t0\t0\t0\t0\t0\tvarWaveP2\tPdet\t0\t0\tODTpowX(DipPowX)\tfreq\tHeatingAmp\t0\tSine\tDetuning\tsingleFreqDet\tDoppCoolDet-DoppCoolSweep\tdopCoolT*1000\r\nbg img\t\tRamp\t1\t10e-6\t1\t1\t0\t0\t0\t1\t1\t0\t0\t1\t1\t0\t0\t0\t1\t1\t0\t0\t0\t0\t0\t0\t0\t0\t0\t0\t1\t0\t0\t0\t1\t0\t0\tplus_zman\tminus_zman\tcompensation\trMOTcurrF\trMOTpow1\tcombAmplitude(combWidthF)\trMOTdelta(-(rMOTbroadDetuningF +combWidthF/2))\t0\t1\t1\t0\t0\t0\t1\t0\t0\tbMOTdelta(MOTdetuning)\tbMOTpow(0.5)\tProbePow\tPdet\tXshim\tYshim\tZshimVar\tODTpowZ(DipPowZ)\t1\t0\t0\t0\t0\t0\t0\t0\t0\t0\t0\t0\t0\t0\t0\t0\t0\t0\t0\t0\t0\tvarWaveP2\tPdet\t0\t0\tODTpowX(DipPowX)\tfreq\tHeatingAmp\t0\tSine\tDetuning\tsingleFreqDet\tDoppCoolDet-DoppCoolSweep\tdopCoolT*1000\r\nbg img\t\tRamp\t0\t2.8e-3\t1\t1\t0\t0\t0\t1\t1\t0\t0\t1\t1\t0\t0\t0\t1\t1\t0\t0\t0\t0\t0\t0\t0\t0\t0\t0\t1\t0\t0\t0\t1\t1\t0\tplus_zman\tminus_zman\tcompensation\trMOTcurrF\trMOTpow1\tcombAmplitude(combWidthF)\trMOTdelta(-(rMOTbroadDetuningF +combWidthF/2))\t0\t1\t1\t0\t0\t0\t1\t1\t1\tbMOTdelta(MOTdetuning)\tbMOTpow(0.5)\tProbePow\tPdet\tXshim\tYshim\tZshimVar\tODTpowZ(DipPowZ)\t1\t0\t0\t0\t0\t0\t0\t0\t0\t0\t0\t0\t0\t0\t0\t0\t0\t0\t0\t0\t0\tvarWaveP2\tPdet\t0\t0\tODTpowX(DipPowX)\tfreq\tHeatingAmp\t0\tSine\tDetuning\tsingleFreqDet\tDoppCoolDet-DoppCoolSweep\tdopCoolT*1000\r\ntransmit img\t\tRamp\t1\t.28\t1\t1\t0\t0\t0\t1\t1\t0\t0\t1\t1\t0\t0\t0\t1\t1\t0\t0\t0\t0\t0\t0\t0\t0\t0\t0\t1\t0\t0\t0\t1\t1\t0\tplus_zman\tminus_zman\tcompensation\trMOTcurrF\trMOTpow1\tcombAmplitude(combWidthF)\trMOTdelta(-(rMOTbroadDetuningF +combWidthF/2))\t0\t1\t1\t0\t0\t0\t1\t1\t1\tbMOTdelta(MOTdetuning)\tbMOTpow(0.5)\tProbePow\tLineRamp(f,Pdet,Pdet2)\tXshim\tYshim\tZshimVar\tODTpowZ(DipPowZ)\t1\t0\t0\t0\t0\t0\t0\t0\t0\t0\t0\t0\t0\t0\t0\t0\t0\t0\t0\t0\t0\tvarWaveP2\tPdet\t0\t0\tODTpowX(DipPowX)\tfreq\tHeatingAmp\t0\tSine\tDetuning\tsingleFreqDet\tDoppCoolDet-DoppCoolSweep\tdopCoolT*1000\r\nalignment\t\tRamp\t1\t.5\t1\t1\t0\t0\t1\t1\t1\t0\t0\t0\t1\t0\t1\t1\t1\t1\t0\t0\t0\t0\t0\t0\t0\t0\t1m\t0\t1\t0\t0\t0\t0\t1\t1\tplus_zman\tminus_zman\tcompensation\tMOTcurrent\trMOTpow1\tcombAmplitude(combWidthI)\trMOTdelta(-(rMOTbroadDetuningI +combWidthI/2))\t0\t1\t0\t1\t1\t0\t1\t1\t1\tbMOTdelta(MOTdetuning)\tbMOTpow(MOTPow)\tProbePow\tPdet2\tXshim\tYshim\tZshim\tODTpowZ(DipPowZ)\t0\t0\t0\t0\t0\t0\t0\t0\t0\t0\t0\t0\t0\t0\t0\t0\t0\t0\t0\t0\t0\tvarWaveP2\tLineRamp(f,Pdet,BlueLaserLockOffset)\t0\t0\tODTpowX(DipPowX)\tfreq\tHeatingAmp\t0\tSine\tDetuning\tsingleFreqDet\tDoppCoolDet-DoppCoolSweep\tdopCoolT*1000\r\n\r\n\r\n"
  in  "Source of Control Data":refnum<k21>="\\\\CONTROL\\VariableLibrary\\CycleDone"
  out "SPE delete path":path=path "C:/Users/Lab/Documents/LightField/LabviewTemp.spe"
  in  "Flea Data Series Name":string="Sr_Flea_Seq"
  in  "Camera Name":T2="Abs XZ"
  in  "Experiment":T3(ring)=enum."Sr"
  in  "Accept parameters from remote system":bool=TRUE
  in  "Flea Magnification":dbl=0.663
  in  "Flea Image direction":enum16{"XY", "XZ"}(ring)=enum."XZ"
  in  "Flea Imaging technique":enum16{"Absorption", "Fluorescence", "RawImage"}(ring)
  in  "Send Flea data to Igor?":bool=TRUE
  out "Command to Igor":string="AutoRunV4(\"Sr_Flea_Seq\",\"C:\\\\Experiment\\\\Data\\\\Flea3_20S4Mtemp.ibw\",\"Sr_PIXIS_Seq\",\"C:\\\\Experiment\\\\Data\\\\PIXIStemp.ibw\") "